vi "python hdf5 speed test.vi"() -> ()   [LabVIEW 2020]
panel:
  out "x-y":u32
  out "data string":string
  in  "small image":bool
  out "return value 2":T1
  out "error out":errorcluster
  out "open error":string
  in  "hdf5 root path":path=path "C:/GEECS/data"
  in  "# shots in scan":i32=1
  out "time per image (ms)":dbl=1.0
  out "write image time (ms)":u32=1
  out "open session  and open_writetime":u32=368
  in  "camera name":string="Camera1"
  in  "Python version":string="3.8"
  in  "module path":path=path "C:/GEECS/Developers Version/source/Axel/openPMD-CCD/openpmd_ccd_labview.py"
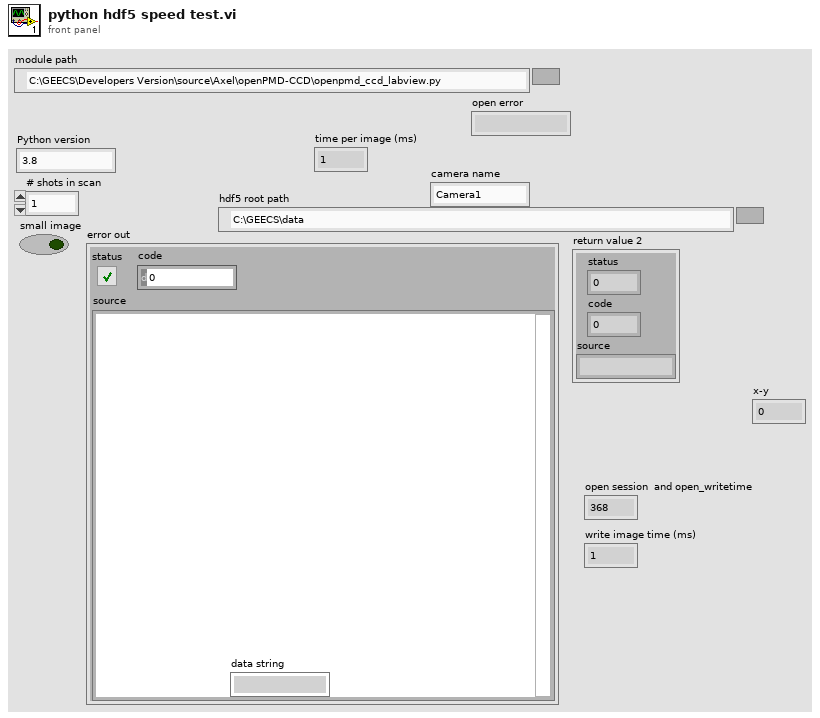
[diagram p1: front panel]
types:
  T1 = cluster{"status":i32, "code":i32, "source":string}
  T2 = enum32{"Map Pixel Pointer", "Unmap Pixel Pointer", "Get Pixels Infos"}
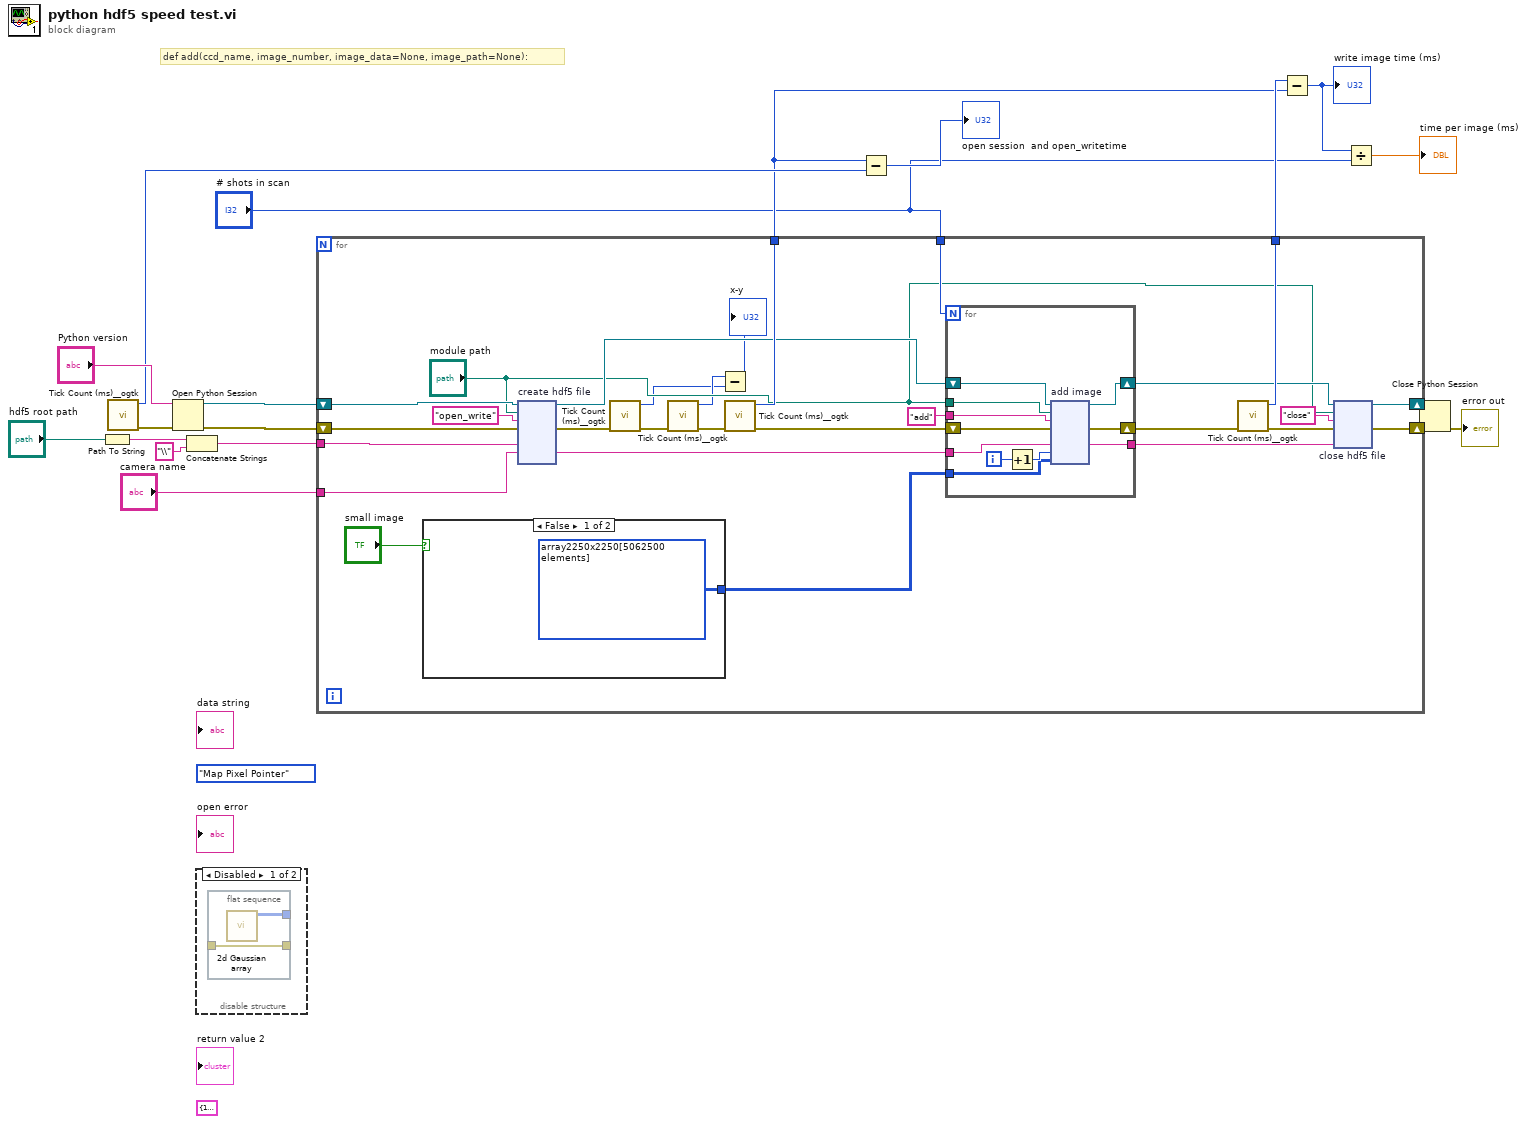
[diagram p0: block diagram]
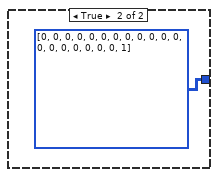
[diagram p2: hidden frame]
diagram:
  (unwired) T2."Map Pixel Pointer" ("Function")
  (unwired) T1 {"status"=1, "code"=1, "source"=""}
  # "def add(ccd_name, image_number, image_data=None, image_path=None):"
  n1 = Path To String(path="hdf5 root path") -> (string=w7:string)
  n2 = call <userlib>:"Tick Count (ms)__ogtk.vi"() -> ("error out"=w17:errorcluster, "millisecond timer value"=w18:u32)  [unwired: 10 in]
  n3 = Open Python Session(python version="Python version", 3:w17) -> (session out=w13:refnum<k35>, error out=w3:errorcluster)  [unwired: 1 in]
  n4 = Concatenate Strings(w7, "\\") -> (w5:string)
  n5 = disable-structure shown="Disabled" {
    frame Disabled {
      n6 = flat-sequence {
        tunnel: [w21] -> _
        tunnel: _ -> [w20]
        tunnel: [w20] -> _
        frame #0 {
          n7 = call "2d Gaussian array.vi"() -> ("Intensity Graph"=w21:u16[][])  [unwired: 11 in]
        }
      }
    }
    frame Enabled {
    }
  }
  n8 = for {
    tunnel: [w47] -> w16
    tunnel: [w46] -> w15
    tunnel: "# shots in scan" -> [w43]
    tunnel: w5 -> [w38]
    tunnel: "camera name" -> [w31]
    shift-right: [w39] -> w9
    shift-left: w13 -> [w45]
    shift-right: [w35] -> w4
    shift-left: w3 -> [w32]
    n9 = case shown="False" "small image" {
      tunnel: [u16[][] array2250x2250[5062500 elements] ("Array") u16[][] [[0, 0, 0, 0, 0], [0, 0, 0, 0, 0], [0, 0, 0, 0, 0], [0, 0, 0, 0, 1]]] -> w23
      frame False {
      }
      frame True {
      }
    }
    n10 = node "create hdf5 file"(w45, "module path", "open_write" ("open h5 function"), w32, w38, w31) -> (w44:refnum<k35>, w25:errorcluster, w37:string)  [unwired: 5 in, 2 out]
    n11 = call <userlib>:"Tick Count (ms)__ogtk.vi"("error in (no error)"=w25) -> ("error out"=w22:errorcluster, "millisecond timer value"=w27:u32)  [unwired: 9 in]
    n12 = call <userlib>:"Tick Count (ms)__ogtk.vi"("error in (no error)"=w22) -> ("error out"=w24:errorcluster, "millisecond timer value"=w28:u32)  [unwired: 9 in]
    n13 = Subtract(x=w28, y=w27) -> (x-y=→"x-y":u32)
    n14 = call <userlib>:"Tick Count (ms)__ogtk.vi"("error in (no error)"=w24) -> ("error out"=w48:errorcluster, "millisecond timer value"=w46:u32)  [unwired: 9 in]
    n15 = for {
      N: w43 -> [_]
      tunnel: "module path" -> [w60]
      tunnel: "add" ("function name") -> [w52]
      tunnel: w37 -> [w55]
      shift-right: [w61] -> w42
      shift-left: w44 -> [w62]
      shift-right: [w58] -> w33
      shift-left: w48 -> [w59]
      tunnel: [w57] -> w36
      tunnel: w23 -> [w53]
      i -> [w56]
      n16 = Increment(x=w56) -> (x+1=w54:i32)
      n17 = node "add image"(w62, w60, w52, w59, w55, w54, w53) -> (w61:refnum<k35>, w58:errorcluster, w57:string)  [unwired: 4 in, 2 out]
    }
    n18 = call <userlib>:"Tick Count (ms)__ogtk.vi"("error in (no error)"=w33) -> ("error out"=w34:errorcluster, "millisecond timer value"=w47:u32)  [unwired: 9 in]
    n19 = node "close hdf5 file"(w42, "module path", "close" ("function name"), w34, w36) -> (w39:refnum<k35>, w35:errorcluster)  [unwired: 3 in, 2 out]
  }
  n20 = Subtract(x=w15, y=w18) -> (x-y=→"open session  and open_writetime":u32)
  n21 = Subtract(x=w16, y=w15) -> (x-y=w12:u32)
  "write image time (ms)" <- w12
  n22 = Divide(x=w12, y="# shots in scan") -> (x/y=→"time per image (ms)":dbl)
  n23 = Close Python Session(session in=w9, error in=w4) -> (11:→"error out":errorcluster)
